vi "ContourPlot v4 IV.vi"() -> ()   [LabVIEW 2020]
uses:
  diff para.ctl
  graph para.ctl
panel:
  in  "Help":bool caption="load data"
  out "smoothed dIV buffer":dbl[][](array[numeric])
  in  "diff para":T1={"x0"=-1.0, "Ic0"=2.0, "h0"=1.0, "y0"=0.0}
  in  "Plot reference":bool caption="load data"
  out "smoothed dIV":dbl[][](array[numeric])
  out "smoothed data":dbl[][](array[numeric])
  in  "smooth n":i32=10
  out "IVdata":dbl[][](array[numeric])
  in  "load data":bool
  out "Status":string="Stopped"
  in  "stop":bool
  in  "Begin":i32=2000
  in  "length":i32=2000
  in  "Contact Resistance":dbl
  in  "Tab Control 2":enum32{"IV plots", "IV smoothed", "dV/dI"}(tab)=enum."dV/dI"
  out "IV Intensity":dbl[][](graph)
  out "IV":cluster{dbl[], "Intensity Graph":dbl[]}(graph)
  in  "Plot contour line":bool
  out "IV smoothed intensity":dbl[][](graph)
  out "Smooth IV":cluster{dbl[], "Intensity Graph":dbl[]}(graph)
  in  "Set diff parameter":bool caption="load data"
  out "dVdI Intensity":dbl[][](graph)
  out "dV/dI":cluster{dbl[], "Intensity Graph":dbl[]}(graph)
  in  "book number":i32=703
  in  "file path":path
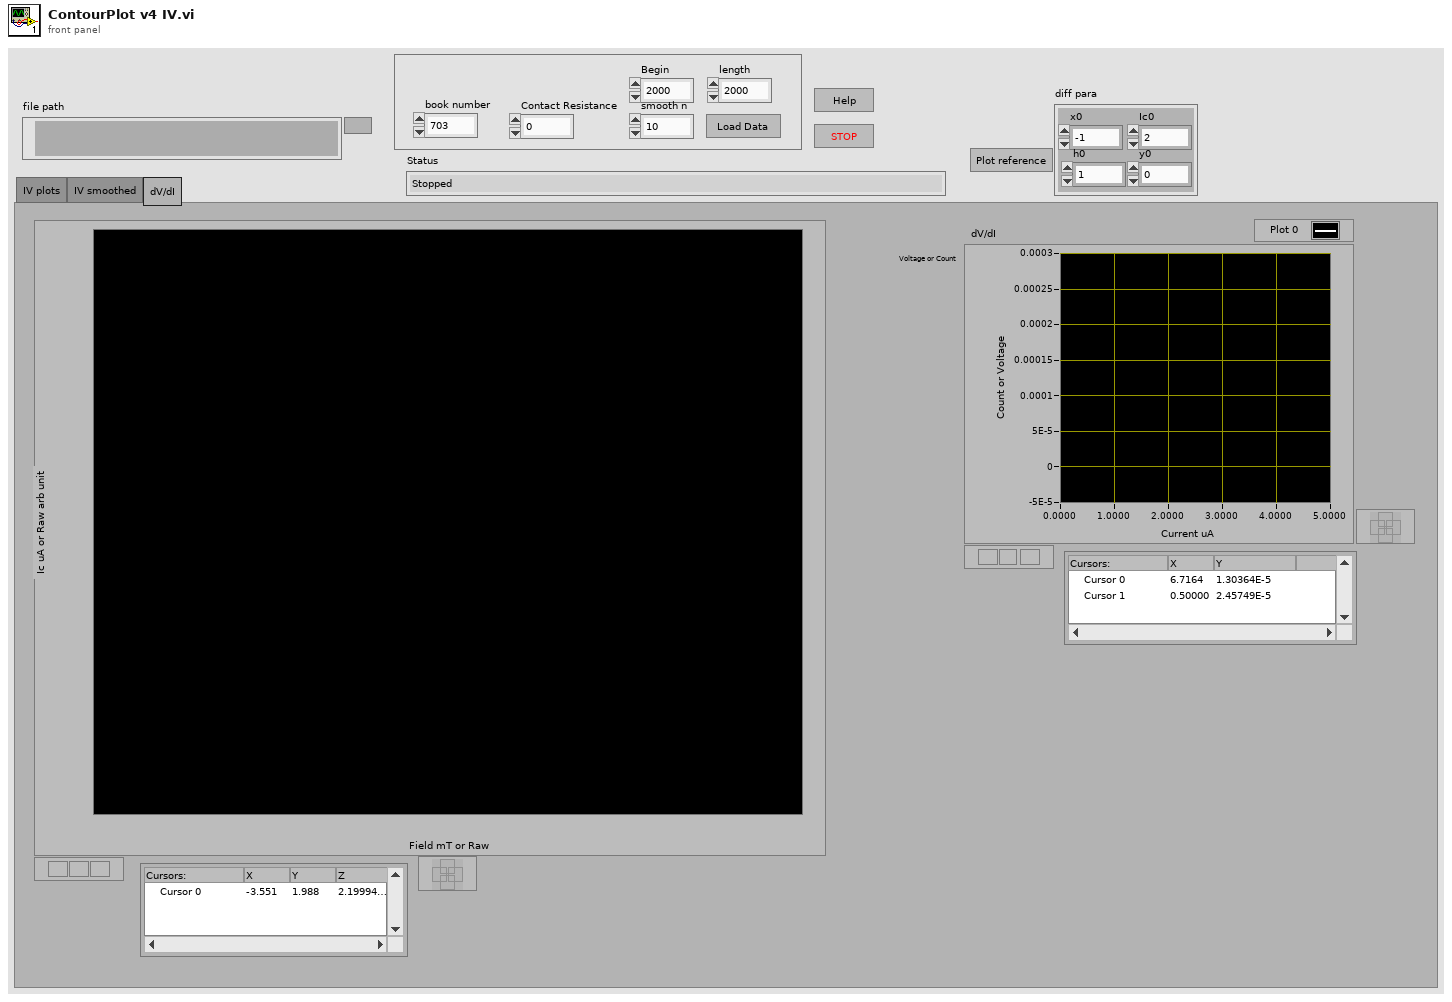
[diagram p1: front panel]
types:
  T1 = typedef "diff para.ctl" = cluster{"x0":dbl, "Ic0":dbl, "h0":dbl, "y0":dbl}
  T2 = typedef "graph para.ctl" = cluster{"x offset":dbl, "y offset":dbl, "x scale":dbl, "y scale":dbl}
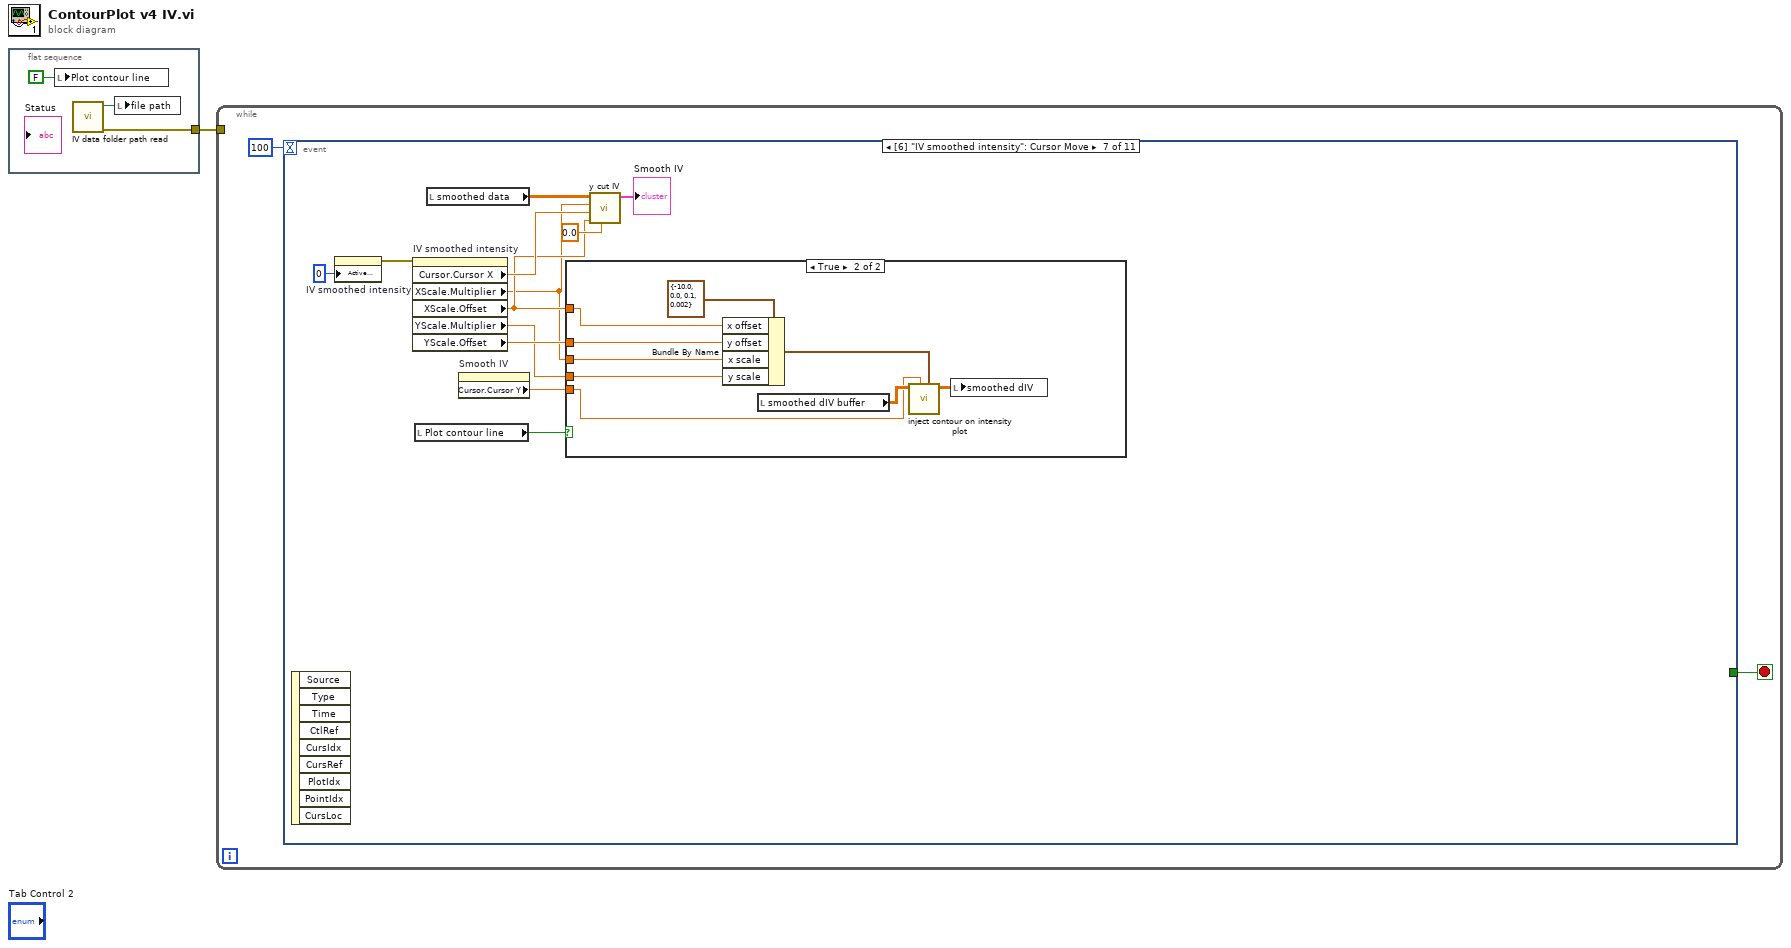
[diagram p0: block diagram]
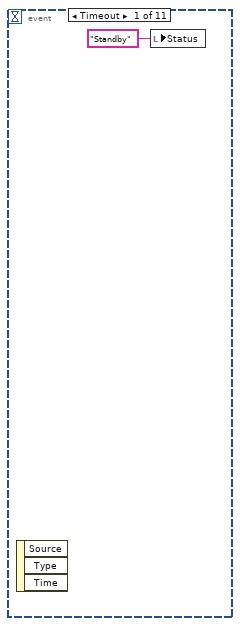
[diagram p2: hidden frame]
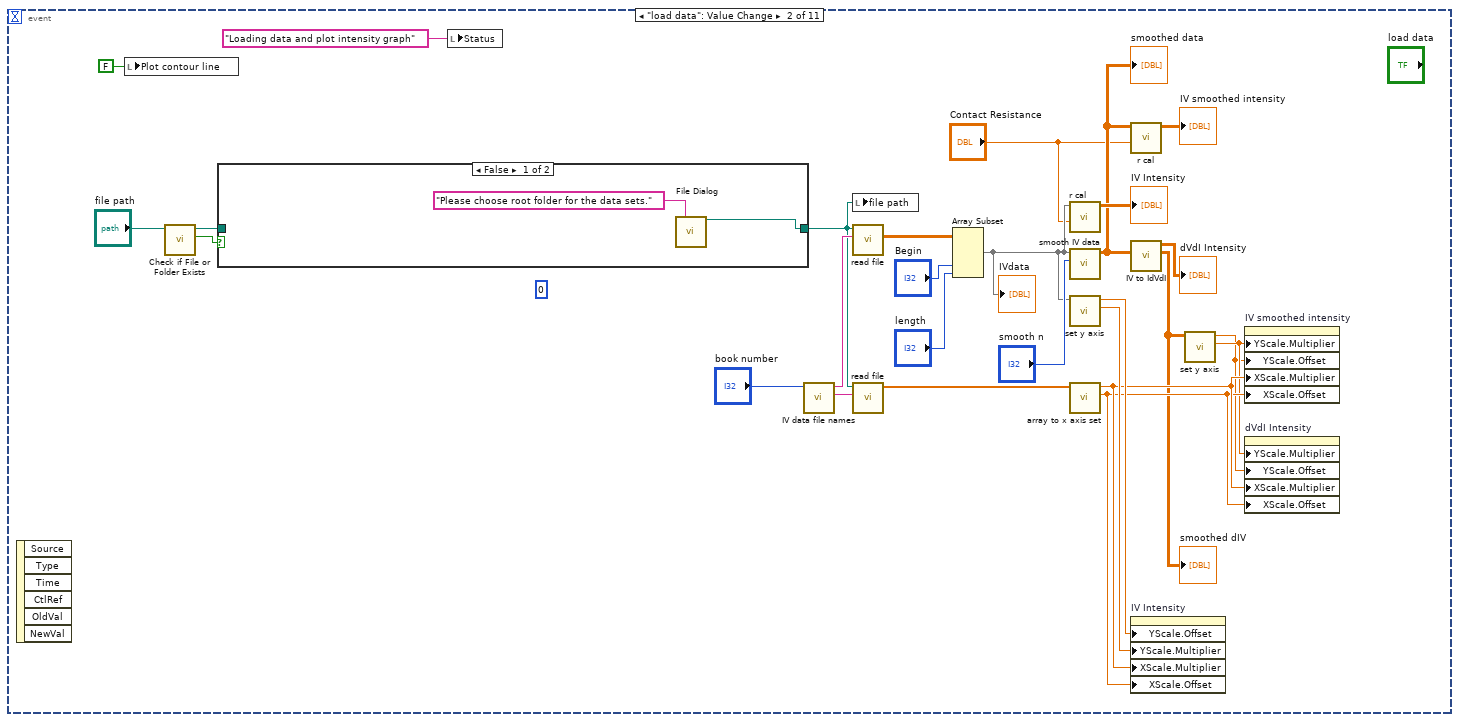
[diagram p3: hidden frame]
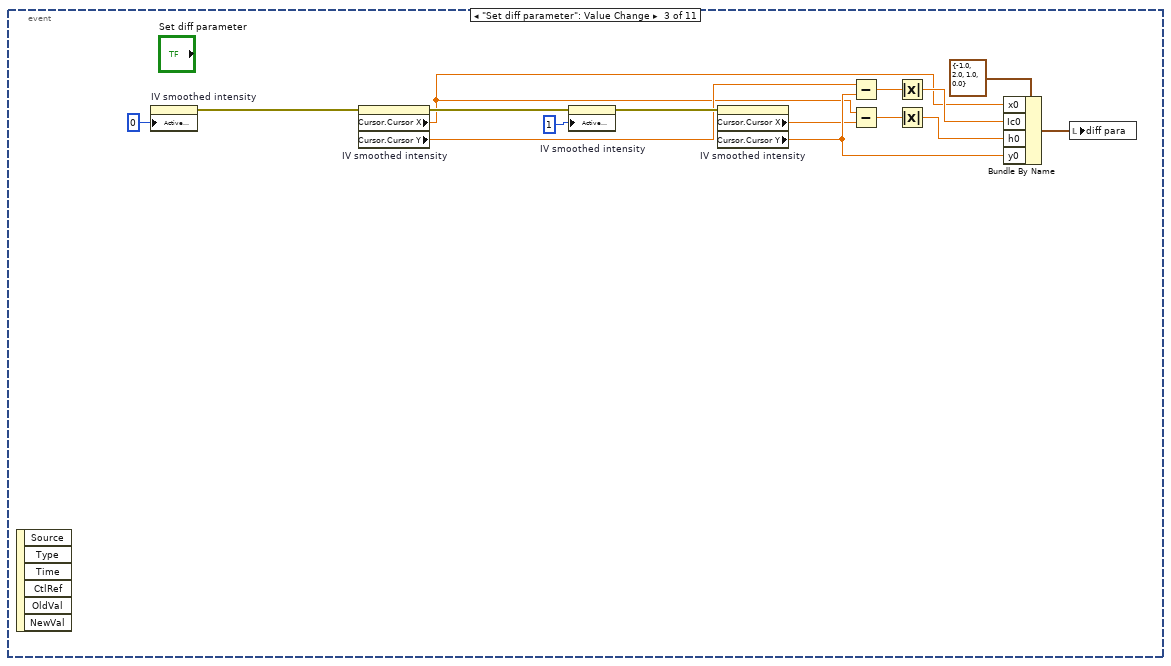
[diagram p5: hidden frame]
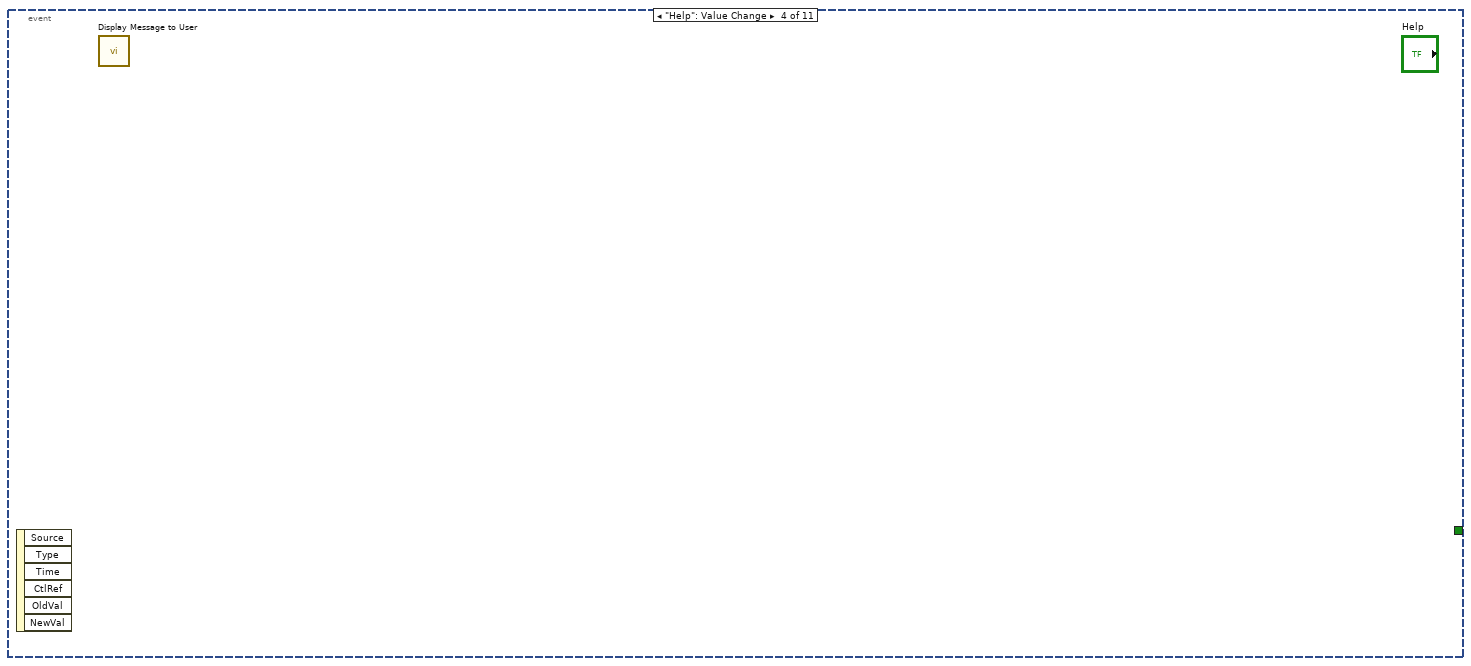
[diagram p6: hidden frame]
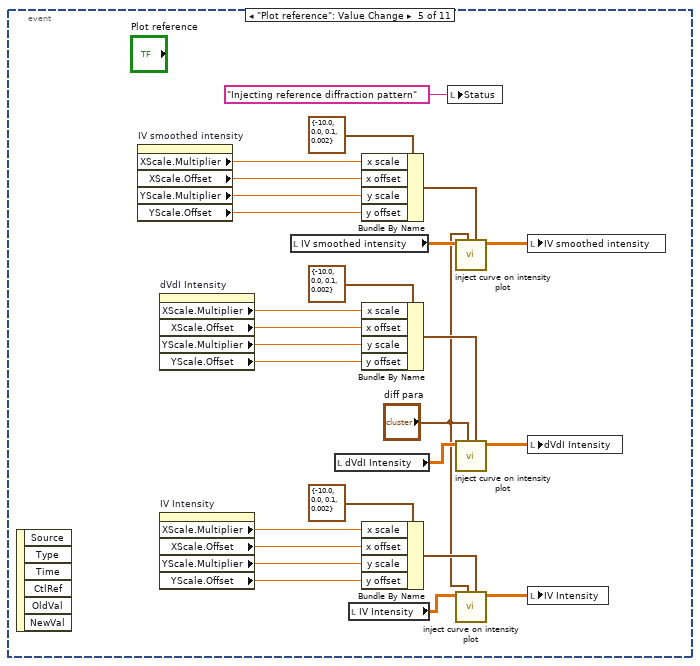
[diagram p7: hidden frame]
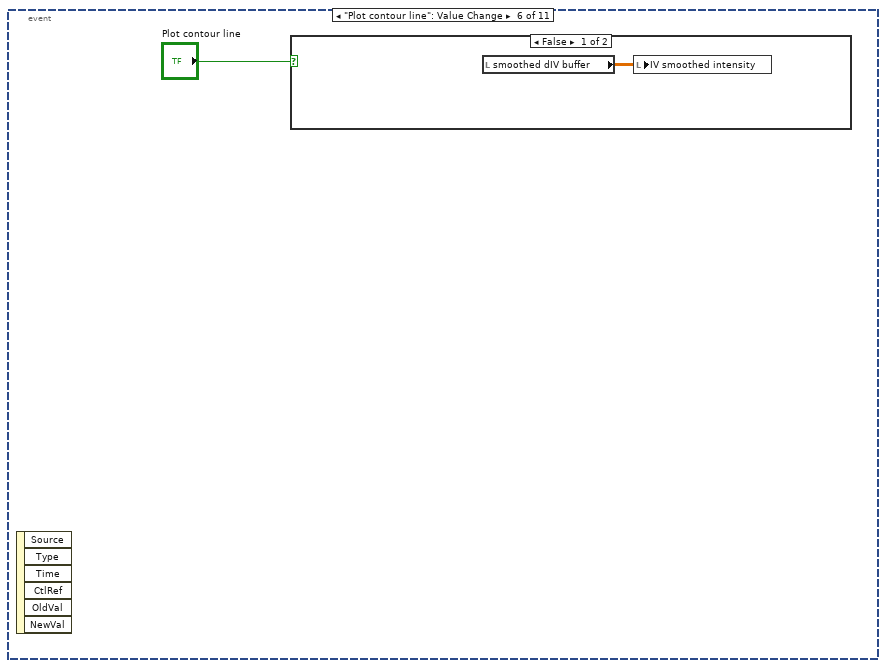
[diagram p8: hidden frame]
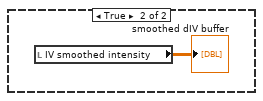
[diagram p9: hidden frame]
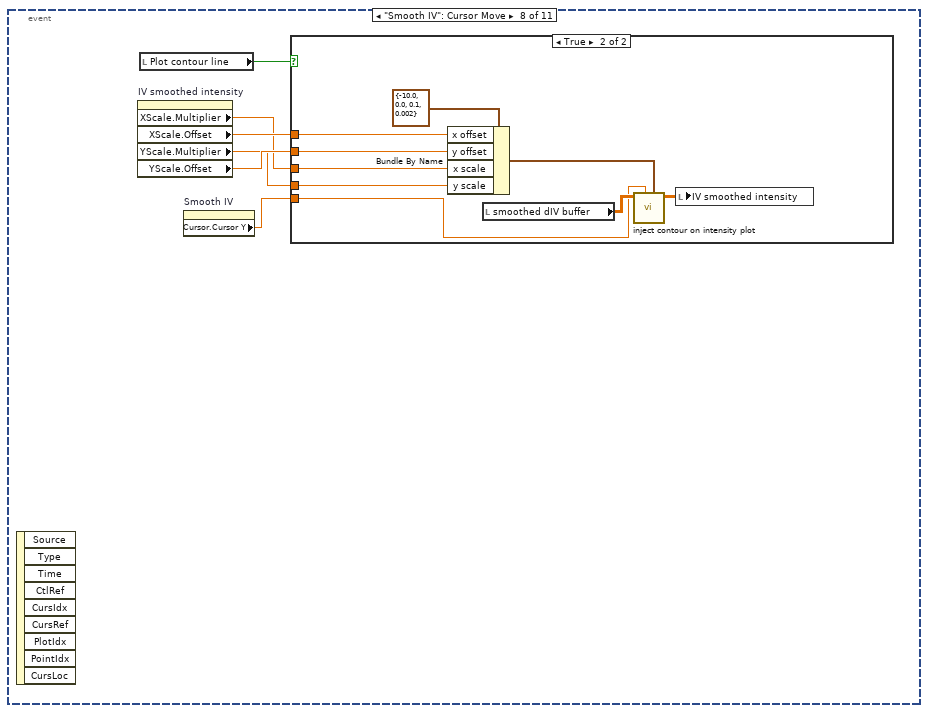
[diagram p11: hidden frame]
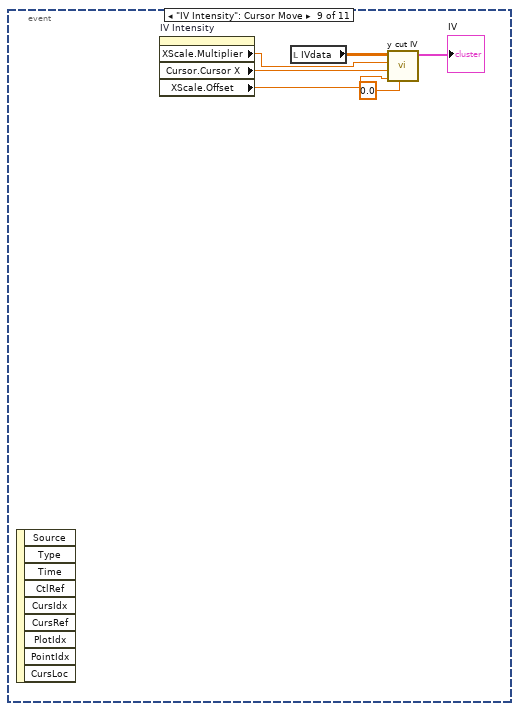
[diagram p13: hidden frame]
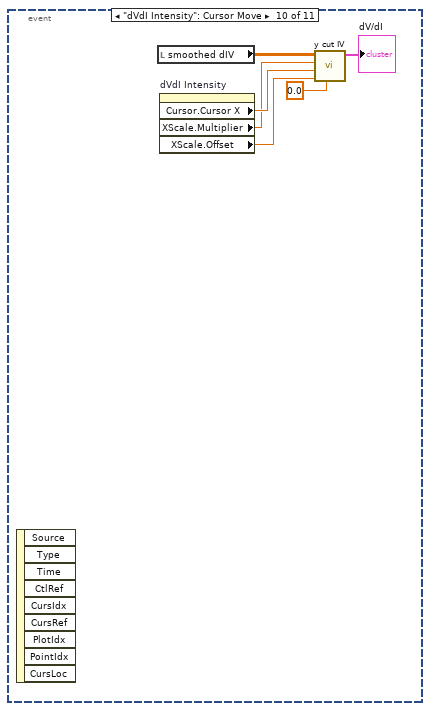
[diagram p14: hidden frame]
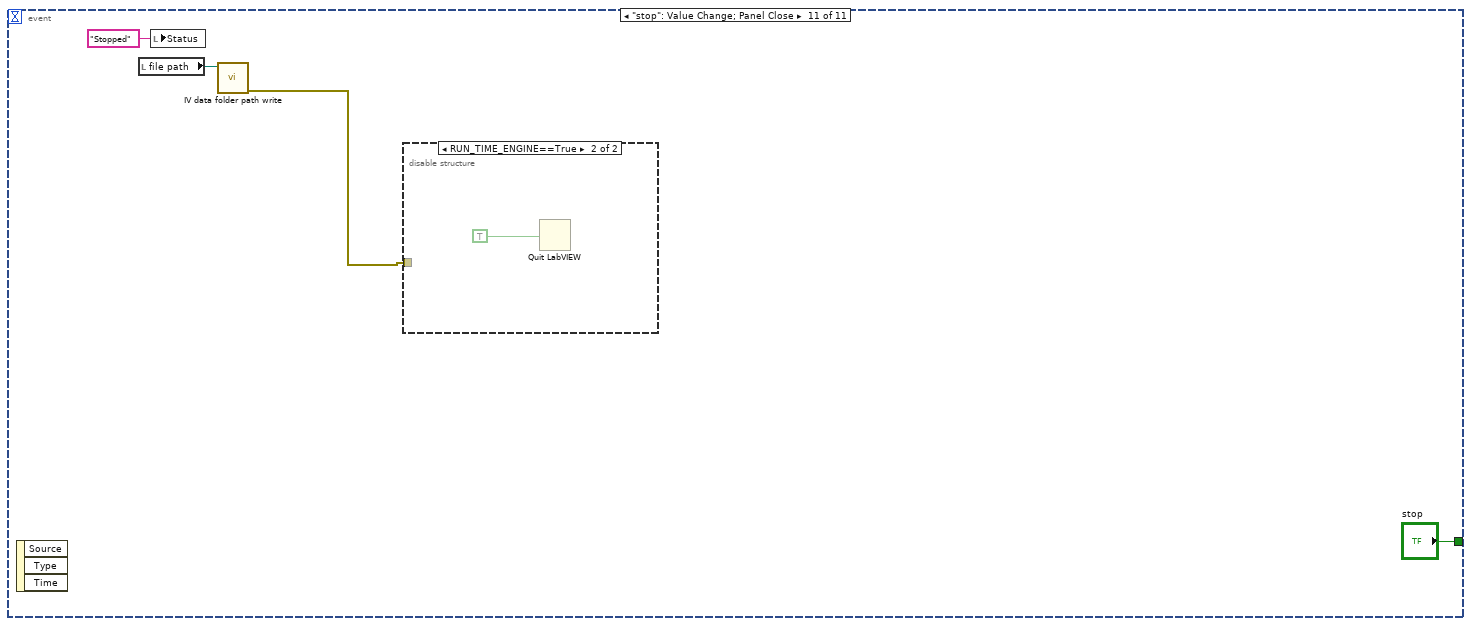
[diagram p15: hidden frame]
diagram:
  n1 = flat-sequence {
    tunnel: [w2] -> w1
    frame #0 {
      n2 = local write "Plot contour line"(FALSE ("Plot contour line")) -> ()
      n3 = call "IV data folder path read.vi"() -> ("error out"=w2:errorcluster, "path"=w3:path)  [unwired: 10 in]
      n4 = local write "file path"(w3) -> ()
    }
  }
  n5 = while {
    tunnel: w1 -> [_]
    stop <- w5 stop-if-true
    n6 = event shown="[6] \"IV smoothed intensity\": Cursor Move" {
      selector: _ -> [_ _ _ _ _ _ _ _ _ _ _]
      dyn-events: _ -> [_ _ _ _ _ _ _ _ _ _ _]
      timeout: 100 -> [_ _ _ _ _ _ _ _ _ _ _]
      tunnel: [_ _ _ _ _ _ _ _ _ _ "stop"] -> w5
      event Timeout {
        n7 = event-data() -> ()  [unwired: 1 in, 3 out]
        n8 = local write "Status"("Standby" ("Status")) -> ()
      }
      event "load data": Value Change {
        (unwired) 0 ("index (row)")
        n9 = event-data() -> ()  [unwired: 1 in, 6 out]
        n10 = local write "Plot contour line"(FALSE ("Plot contour line")) -> ()
        n11 = call <vilib>:"Check if File or Folder Exists.vi"("path"="file path") -> ("file or folder exists?"=w10:bool, "dup path"=w9:path)  [unwired: 8 in, 1 out]
        n12 = case shown="False" w10 {
          tunnel: [w35 w37] -> w8
          tunnel: w9 -> [_ w37]
          frame False {
            n13 = call "File Dialog"("prompt"="Please choose root folder for the data sets.") -> ("selected path"=w35:path)  [unwired: 11 in, 3 out]
          }
          frame True {
          }
        }
        n14 = local write "Status"("Loading data and plot intensity graph" ("Status")) -> ()
        n15 = call "IV data file names.vi"("book number"="book number") -> ("Field"=w33:string, "IV"=w32:string)  [unwired: 8 in, 1 out]
        n16 = local write "file path"(w8) -> ()
        n17 = call "read file.vi"("file name"=w32, "file path (dialog if empty)"=w8) -> ("2d data"=w25:dbl[][])  [unwired: 8 in, 1 out]
        n18 = call "read file.vi"("file name"=w33, "file path (dialog if empty)"=w8) -> ("1d Data"=w24:dbl[])  [unwired: 8 in, 1 out]
        n19 = Array Subset(array=w25, index (col)="Begin", length (col)="length") -> (w21:dbl[][])  [unwired: 2 in]
        "IVdata" <- w21
        n20 = call "r cal.vi"("Contact Resistance"="Contact Resistance", "Array in"=w21) -> ("Array out"=→"IV Intensity":dbl[][])  [unwired: 9 in]
        n21 = call "smooth IV data.vi"("smooth n"="smooth n", "Array in"=w21) -> ("Array out"=w20:dbl[][])  [unwired: 9 in]
        "smoothed data" <- w20
        n22 = call "set y axis.vi"("Array"=w21) -> ("y multi"=w31:dbl, "y offset"=w30:dbl)  [unwired: 9 in]
        n23 = call "array to x axis set.vi"("1d Data"=w24) -> ("offset"=w16:dbl, "multiplier"=w17:dbl)  [unwired: 9 in]
        n24 = call "r cal.vi"("Contact Resistance"="Contact Resistance", "Array in"=w20) -> ("Array out"=→"IV smoothed intensity":dbl[][])  [unwired: 9 in]
        n25 = call "IV to IdVdI.vi"("Array in"=w20) -> ("Array"=w15:dbl[][], "Array 2"=→"dVdI Intensity":dbl[][])  [unwired: 9 in]
        "smoothed dIV" <- w15
        n26 = property on="IV Intensity" class="IntGraph (strict)"("YScale.Offset"=w30, "YScale.Multiplier"=w31, "XScale.Multiplier"=w17, "XScale.Offset"=w16) -> ()  [unwired: 2 in, 2 out]
        n27 = call "set y axis.vi"("Array"=w15) -> ("y multi"=w14:dbl, "y offset"=w13:dbl)  [unwired: 9 in]
        n28 = property on="IV smoothed intensity" class="IntGraph (strict)"("YScale.Multiplier"=w14, "YScale.Offset"=w13, "XScale.Multiplier"=w17, "XScale.Offset"=w16) -> ()  [unwired: 2 in, 2 out]
        n29 = property on="dVdI Intensity" class="IntGraph (strict)"("YScale.Multiplier"=w14, "YScale.Offset"=w13, "XScale.Multiplier"=w17, "XScale.Offset"=w16) -> ()  [unwired: 2 in, 2 out]
      }
      event "Set diff parameter": Value Change {
        n30 = event-data() -> ()  [unwired: 1 in, 6 out]
        n31 = property on="IV smoothed intensity" class="IntGraph (strict)"("Active Cursor"=u32 0) -> (error out=w52:errorcluster)  [unwired: 2 in, 1 out]
        n32 = property on="IV smoothed intensity" class="IntGraph (strict)"(error in=w52) -> (error out=w49:errorcluster, "Cursor.Cursor X"=w41:dbl, "Cursor.Cursor Y"=w45:dbl)  [unwired: 1 in, 1 out]
        n33 = property on="IV smoothed intensity" class="IntGraph (strict)"(error in=w49, "Active Cursor"=u32 1) -> (error out=w48:errorcluster)  [unwired: 1 in, 1 out]
        n34 = property on="IV smoothed intensity" class="IntGraph (strict)"(error in=w48) -> ("Cursor.Cursor X"=w40:dbl, "Cursor.Cursor Y"=w44:dbl)  [unwired: 1 in, 2 out]
        n35 = Subtract(x=w45, y=w44) -> (x-y=w43:dbl)
        n36 = Subtract(x=w41, y=w40) -> (x-y=w39:dbl)
        n37 = Absolute Value(x=w43) -> (abs(x)=w42:dbl)
        n38 = Absolute Value(x=w39) -> (abs(x)=w38:dbl)
        n39 = Bundle By Name(cluster=T1 {"x0"=-1.0, "Ic0"=2.0, "h0"=1.0, "y0"=0.0} ("diff para"), "x0"=w41, "Ic0"=w42, "h0"=w38, "y0"=w44) -> (w47:T1)
        n40 = local write "diff para"(w47) -> ()
      }
      event "Help": Value Change {
        n41 = event-data() -> ()  [unwired: 1 in, 6 out]
        n42 = call "Display Message to User"() -> ()  [unwired: 10 in, 2 out]
      }
      event "Plot reference": Value Change {
        n43 = event-data() -> ()  [unwired: 1 in, 6 out]
        n44 = property on="IV smoothed intensity" class="IntGraph (strict)"() -> ("XScale.Multiplier"=w64:dbl, "XScale.Offset"=w63:dbl, "YScale.Multiplier"=w62:dbl, "YScale.Offset"=w61:dbl)  [unwired: 2 in, 2 out]
        n45 = property on="dVdI Intensity" class="IntGraph (strict)"() -> ("XScale.Multiplier"=w58:dbl, "XScale.Offset"=w57:dbl, "YScale.Multiplier"=w56:dbl, "YScale.Offset"=w55:dbl)  [unwired: 2 in, 2 out]
        n46 = property on="IV Intensity" class="IntGraph (strict)"() -> ("XScale.Multiplier"=w76:dbl, "XScale.Offset"=w75:dbl, "YScale.Multiplier"=w74:dbl, "YScale.Offset"=w73:dbl)  [unwired: 2 in, 2 out]
        n47 = local read "IV smoothed intensity"() -> (w65:dbl[][])
        n48 = local read "dVdI Intensity"() -> (w59:dbl[][])
        n49 = local read "IV Intensity"() -> (w78:dbl[][])
        n50 = Bundle By Name(cluster=T2 {"x offset"=-10.0, "y offset"=0.0, "x scale"=0.1, "y scale"=0.002} ("graph para"), "x scale"=w64, "x offset"=w63, "y scale"=w62, "y offset"=w61) -> (w68:T2)
        n51 = Bundle By Name(cluster=T2 {"x offset"=-10.0, "y offset"=0.0, "x scale"=0.1, "y scale"=0.002} ("graph para"), "x scale"=w58, "x offset"=w57, "y scale"=w56, "y offset"=w55) -> (w66:T2)
        n52 = Bundle By Name(cluster=T2 {"x offset"=-10.0, "y offset"=0.0, "x scale"=0.1, "y scale"=0.002} ("graph para"), "x scale"=w76, "x offset"=w75, "y scale"=w74, "y offset"=w73) -> (w72:T2)
        n53 = local write "Status"("Injecting reference diffraction pattern" ("Status")) -> ()
        n54 = call "inject curve on intensity plot.vi"("graph para"=w68, "diff para"="diff para", "IV Intensity"=w65) -> ("IV Intensity 2"=w60:dbl[][])  [unwired: 8 in]
        n55 = call "inject curve on intensity plot.vi"("graph para"=w66, "diff para"="diff para", "IV Intensity"=w59) -> ("IV Intensity 2"=w53:dbl[][])  [unwired: 8 in]
        n56 = call "inject curve on intensity plot.vi"("graph para"=w72, "diff para"="diff para", "IV Intensity"=w78) -> ("IV Intensity 2"=w71:dbl[][])  [unwired: 8 in]
        n57 = local write "IV smoothed intensity"(w60) -> ()
        n58 = local write "dVdI Intensity"(w53) -> ()
        n59 = local write "IV Intensity"(w71) -> ()
      }
      event "Plot contour line": Value Change {
        n60 = event-data() -> ()  [unwired: 1 in, 6 out]
        n61 = case shown="False" "Plot contour line" {
          frame False {
            n62 = local read "smoothed dIV buffer"() -> (w80:dbl[][])
            n63 = local write "IV smoothed intensity"(w80) -> ()
          }
          frame True {
            n64 = local read "IV smoothed intensity"() -> (→"smoothed dIV buffer":dbl[][])
          }
        }
      }
      event "IV smoothed intensity": Cursor Move {
        n65 = event-data() -> ()  [unwired: 1 in, 9 out]
        n66 = property on="IV smoothed intensity" class="IntGraph (strict)"("Active Cursor"=u32 0) -> (error out=w82:errorcluster)  [unwired: 2 in, 1 out]
        n67 = property on="IV smoothed intensity" class="IntGraph (strict)"(error in=w82) -> ("Cursor.Cursor X"=w90:dbl, "XScale.Multiplier"=w86:dbl, "XScale.Offset"=w88:dbl, "YScale.Multiplier"=w85:dbl, "YScale.Offset"=w87:dbl)  [unwired: 1 in, 2 out]
        n68 = local read "Plot contour line"() -> (w89:bool)
        n69 = local read "smoothed data"() -> (w93:dbl[][])
        n70 = property on="Smooth IV" class="XYGraph (strict)"() -> ("Cursor.Cursor Y"=w84:dbl)  [unwired: 2 in, 2 out]
        n71 = case shown="True" w89 {
          tunnel: w84 -> [_ w100]
          tunnel: w88 -> [_ w98]
          tunnel: w87 -> [_ w97]
          tunnel: w86 -> [_ w96]
          tunnel: w85 -> [_ w95]
          frame False {
          }
          frame True {
            n72 = Bundle By Name(cluster=T2 {"x offset"=-10.0, "y offset"=0.0, "x scale"=0.1, "y scale"=0.002} ("graph para"), "x offset"=w98, "y offset"=w97, "x scale"=w96, "y scale"=w95) -> (w94:T2)
            n73 = local read "smoothed dIV buffer"() -> (w102:dbl[][])
            n74 = call "inject contour on intensity plot.vi"("graph para"=w94, "Threshold"=w100, "IV Intensity"=w102) -> ("IV Intensity output"=w101:dbl[][])  [unwired: 6 in, 2 out]
            n75 = local write "smoothed dIV"(w101) -> ()
          }
        }
        n76 = call "y cut IV.vi"("Contact Resistance"=0.0, "x offset"=w88, "x pos"=w90, "scale"=w86, "Data"=w93) -> ("IV"=→"Smooth IV":cluster{"Data":dbl[], dbl[]})  [unwired: 4 in, 2 out]
      }
      event "Smooth IV": Cursor Move {
        n77 = event-data() -> ()  [unwired: 1 in, 9 out]
        n78 = property on="IV smoothed intensity" class="IntGraph (strict)"() -> ("XScale.Multiplier"=w105:dbl, "XScale.Offset"=w107:dbl, "YScale.Multiplier"=w104:dbl, "YScale.Offset"=w106:dbl)  [unwired: 2 in, 2 out]
        n79 = local read "Plot contour line"() -> (w108:bool)
        n80 = property on="Smooth IV" class="XYGraph (strict)"() -> ("Cursor.Cursor Y"=w103:dbl)  [unwired: 2 in, 2 out]
        n81 = case shown="True" w108 {
          tunnel: w103 -> [_ w115]
          tunnel: w107 -> [_ w113]
          tunnel: w106 -> [_ w112]
          tunnel: w105 -> [_ w111]
          tunnel: w104 -> [_ w110]
          frame False {
          }
          frame True {
            n82 = Bundle By Name(cluster=T2 {"x offset"=-10.0, "y offset"=0.0, "x scale"=0.1, "y scale"=0.002} ("graph para"), "x offset"=w113, "y offset"=w112, "x scale"=w111, "y scale"=w110) -> (w109:T2)
            n83 = local read "smoothed dIV buffer"() -> (w117:dbl[][])
            n84 = call "inject contour on intensity plot.vi"("graph para"=w109, "Threshold"=w115, "IV Intensity"=w117) -> ("IV Intensity output"=w116:dbl[][])  [unwired: 6 in, 2 out]
            n85 = local write "IV smoothed intensity"(w116) -> ()
          }
        }
      }
      event "IV Intensity": Cursor Move {
        n86 = event-data() -> ()  [unwired: 1 in, 9 out]
        n87 = property on="IV Intensity" class="IntGraph (strict)"() -> ("XScale.Multiplier"=w120:dbl, "Cursor.Cursor X"=w121:dbl, "XScale.Offset"=w122:dbl)  [unwired: 2 in, 2 out]
        n88 = local read "IVdata"() -> (w119:dbl[][])
        n89 = call "y cut IV.vi"("Contact Resistance"=0.0, "x offset"=w122, "x pos"=w121, "scale"=w120, "Data"=w119) -> ("IV"=→"IV":cluster{"Data":dbl[], dbl[]})  [unwired: 4 in, 2 out]
      }
      event "dVdI Intensity": Cursor Move {
        n90 = event-data() -> ()  [unwired: 1 in, 9 out]
        n91 = local read "smoothed dIV"() -> (w129:dbl[][])
        n92 = property on="dVdI Intensity" class="IntGraph (strict)"() -> ("Cursor.Cursor X"=w127:dbl, "XScale.Multiplier"=w126:dbl, "XScale.Offset"=w125:dbl)  [unwired: 2 in, 2 out]
        n93 = call "y cut IV.vi"("Contact Resistance"=0.0, "x offset"=w125, "x pos"=w127, "scale"=w126, "Data"=w129) -> ("IV"=→"dV/dI":cluster{"Data":dbl[], dbl[]})  [unwired: 4 in, 2 out]
      }
      event "stop": Value Change; Panel Close {
        n94 = event-data() -> ()  [unwired: 1 in, 3 out]
        n95 = local read "file path"() -> (w131:path)
        n96 = local write "Status"("Stopped" ("Status")) -> ()
        n97 = call "IV data folder path write.vi"("Path"=w131) -> ("error out"=w130:errorcluster)  [unwired: 10 in]
        n98 = disable-structure shown="RUN_TIME_ENGINE==True" {
          disable-tunnel: w130 -> [_ _]
          frame condition #0 (active) {
          }
          frame condition #1 {
            n99 = Quit LabVIEW(quit? (T)=TRUE) -> ()
          }
        }
      }
    }
  }
